vi "Project-SmartHome.vi"() -> ()   [LabVIEW 2013]
uses:
  <vilib>/regexp/Match Regular Expression.xnode
panel:
  in  "Back":bool
  out "Numeric":dbl
  in  "Tab Control 25":enum32{"Page 1", "Page 2"}(tab)
  in  "Back 22":bool
  in  "edit":bool
  out "Table Control":string[][](table)
  in  "String":string
  in  "flag 8":u16(ring) items=["Admin", "User"]
  in  "String":string
  in  "String":string
  in  "delete":bool
  in  "add":bool
  out "channel":dbl
  out "URL":string="C:\\Users\\kiat\\Downloads\\asd.mp4"
  in  "Tab Control 24":enum32{"Page 1", "Page 2"}(tab)
  in  "Back 21":bool
  in  "WindowsMediaPlayer":refnum<k7>(container)
  in  "backward":bool
  in  "foward":bool
  in  "pause":bool
  in  "stop":bool
  in  "flag 7":u16(ring) items=["1", "2", "3"]
  in  "play":bool
  in  "?":dbl(slide) scale=0.0..100.0
  in  "Tab Control 23":enum32{"Page 1", "Page 2"}(tab)
  in  "Back 19":bool
  in  "?":bool
  in  "String":string
  in  "?":bool
  in  "?":dbl(slide) scale=16.0..27.0
  in  "Tab Control 22":enum32{"Page 1", "Page 2"}(tab)
  in  "Back 18":bool
  in  "?":bool
  in  "String":string
  in  "?":bool
  in  "?":dbl(slide) scale=16.0..27.0
  in  "Tab Control 21":enum32{"Page 1", "Page 2"}(tab)
  in  "Back 20":bool
  in  "?":bool
  in  "String":string
  in  "?":bool
  in  "?":dbl(slide) scale=16.0..27.0
  in  "Tab Control 19":enum32{"Page 1", "Page 2"}(tab)
  in  "Back 17":bool
  in  "?":bool
  in  "?":bool
  in  "?":bool
  in  "Tab Control 18":enum32{"Page 1", "Page 2"}(tab)
  in  "Back 12":bool
  in  "?":bool
  in  "start hour 3":u16(ring) items=["1", "2", "3", "4", "5", "6", "7", "8", "9", "10", "11", "12"]
  in  "flag 6":u16(ring) items=["AM", "PM"]
  in  "start min 3":u16(ring) items=["0", "1", "2", "3", "4", "5", "6", "7", "8", "9", "10", "11", "12", "13", "14", "15", "16", "17", "18", "19", "20", "21", "22", "23", "24", "25", "26", "27", "28", "29", "30", "31", "32", "33", "34", "35", "36", "37", "38", "39", "40", "41", "42", "43", "44", "45", "46", "47", "48", "49", "50", "51", "52", "53", "54", "55", "56", "57", "58", "59"]
  in  "end hour 3":u16(ring) items=["1", "2", "3", "4", "5", "6", "7", "8", "9", "10", "11", "12"]
  in  "end min 3":u16(ring) items=["0", "1", "2", "3", "4", "5", "6", "7", "8", "9", "10", "11", "12", "13", "14", "15", "16", "17", "18", "19", "20", "21", "22", "23", "24", "25", "26", "27", "28", "29", "30", "31", "32", "33", "34", "35", "36", "37", "38", "39", "40", "41", "42", "43", "44", "45", "46", "47", "48", "49", "50", "51", "52", "53", "54", "55", "56", "57", "58", "59"]
  in  "flag 5":u16(ring) items=["AM", "PM"]
  in  "String":string
  in  "?":bool
  in  "?":dbl(slide) scale=0.0..4.0
  in  "Tab Control 17":enum32{"Page 1", "Page 2"}(tab)
  in  "Back 11":bool
  in  "flag 3":u16(ring) items=["AM", "PM"]
  in  "end min 2":u16(ring) items=["0", "1", "2", "3", "4", "5", "6", "7", "8", "9", "10", "11", "12", "13", "14", "15", "16", "17", "18", "19", "20", "21", "22", "23", "24", "25", "26", "27", "28", "29", "30", "31", "32", "33", "34", "35", "36", "37", "38", "39", "40", "41", "42", "43", "44", "45", "46", "47", "48", "49", "50", "51", "52", "53", "54", "55", "56", "57", "58", "59"]
  in  "end hour 2":u16(ring) items=["1", "2", "3", "4", "5", "6", "7", "8", "9", "10", "11", "12"]
  in  "start min 2":u16(ring) items=["0", "1", "2", "3", "4", "5", "6", "7", "8", "9", "10", "11", "12", "13", "14", "15", "16", "17", "18", "19", "20", "21", "22", "23", "24", "25", "26", "27", "28", "29", "30", "31", "32", "33", "34", "35", "36", "37", "38", "39", "40", "41", "42", "43", "44", "45", "46", "47", "48", "49", "50", "51", "52", "53", "54", "55", "56", "57", "58", "59"]
  in  "flag 4":u16(ring) items=["AM", "PM"]
  in  "start hour 2":u16(ring) items=["1", "2", "3", "4", "5", "6", "7", "8", "9", "10", "11", "12"]
  in  "?":bool
  in  "String":string
  in  "?":bool
  in  "?":dbl(slide) scale=0.0..4.0
  in  "Tab Control 16":enum32{"Page 1", "Page 2"}(tab)
  in  "Back 9":bool
  in  "?":bool
  in  "?":bool
  in  "?":bool
  in  "Tab Control 15":enum32{"Page 1", "Page 2"}(tab)
  in  "Back 16":bool
  in  "OK Button 32":bool
  in  "OK Button 31":bool
  in  "?":bool
  in  "Tab Control 14":enum32{"Page 1", "Page 2"}(tab)
  in  "Back 15":bool
  in  "OK Button 27":bool
  in  "OK Button 26":bool
  in  "OK Button 25":bool
  in  "?":bool
  in  "Tab Control 13":enum32{"Page 1", "Page 2"}(tab)
  in  "Back 14":bool
  in  "OK Button 24":bool
  in  "OK Button 23":bool
  in  "OK Button 22":bool
  in  "OK Button 21":bool
  in  "OK Button 20":bool
  in  "OK Button 19":bool
  in  "?":bool
  in  "Tab Control 12":enum32{"Page 1", "Page 2"}(tab)
  in  "Back 13":bool
  in  "?":bool
  in  "?":bool
  in  "?":bool
  in  "Tab Control 11":enum32{"Page 1", "Page 2"}(tab)
  in  "Back 10":bool
  in  "flag":u16(ring) items=["AM", "PM"]
  in  "end min 1":u16(ring) items=["0", "1", "2", "3", "4", "5", "6", "7", "8", "9", "10", "11", "12", "13", "14", "15", "16", "17", "18", "19", "20", "21", "22", "23", "24", "25", "26", "27", "28", "29", "30", "31", "32", "33", "34", "35", "36", "37", "38", "39", "40", "41", "42", "43", "44", "45", "46", "47", "48", "49", "50", "51", "52", "53", "54", "55", "56", "57", "58", "59"]
  in  "end hour 1":u16(ring) items=["1", "2", "3", "4", "5", "6", "7", "8", "9", "10", "11", "12"]
  in  "start min 1":u16(ring) items=["0", "1", "2", "3", "4", "5", "6", "7", "8", "9", "10", "11", "12", "13", "14", "15", "16", "17", "18", "19", "20", "21", "22", "23", "24", "25", "26", "27", "28", "29", "30", "31", "32", "33", "34", "35", "36", "37", "38", "39", "40", "41", "42", "43", "44", "45", "46", "47", "48", "49", "50", "51", "52", "53", "54", "55", "56", "57", "58", "59"]
  in  "flag 2":u16(ring) items=["AM", "PM"]
  in  "start hour 1":u16(ring) items=["1", "2", "3", "4", "5", "6", "7", "8", "9", "10", "11", "12"]
  in  "?":bool
  in  "String":string
  in  "?":bool
  in  "?":dbl(slide) scale=0.0..4.0
  in  "Tab Control 10":enum32{"Page 1", "Page 2"}(tab)
  in  "Tab Control 9":enum32{"Page 1", "Page 2"}(tab)
  in  "Back 8":bool
  in  "OK Button 18":bool
  in  "?":bool
  in  "Tab Control 8":enum32{"Page 1", "Page 2"}(tab)
  in  "Back 7":bool
  in  "OK Button 17":bool
  in  "?":bool
  in  "Tab Control 7":enum32{"Page 1", "Page 2"}(tab)
  in  "Back 6":bool
  in  "OK Button 16":bool
  in  "?":bool
  in  "Tab Control 6":enum32{"Page 1", "Page 2"}(tab)
  in  "Back 5":bool
  in  "OK Button 15":bool
  in  "?":bool
  in  "Tab Control 5":enum32{"Page 1", "Page 2"}(tab)
  in  "Back 4":bool
  in  "OK Button 14":bool
  in  "OK Button 13":bool
  in  "OK Button 12":bool
  in  "OK Button 11":bool
  in  "?":bool
  in  "Tab Control 4":enum32{"Page 1", "Page 2"}(tab)
  in  "Back 3":bool
  in  "OK Button 10":bool
  in  "OK Button 9":bool
  in  "OK Button 8":bool
  in  "OK Button 7":bool
  in  "OK Button 6":bool
  in  "OK Button 5":bool
  in  "?":bool
  in  "stop":bool
  in  "Tab Control 3":enum32{"Page 1", "Page 2"}(tab)
  in  "Back 2":bool
  in  "?":bool
  in  "?":bool
  in  "?":bool
  in  "?":bool
  in  "?":bool
  in  "?":bool
  in  "Tab Control 2":enum32{"Page 1"}(tab)
  in  "OK Button 3":bool
  in  "?":bool
  in  "?":bool
  in  "?":bool
  in  "?":bool
  in  "?":bool
  in  "?":bool
  in  "Tab Control":enum32{"Page 1", "Page 2"}(tab)
  in  "String 2":string caption="String"
  in  "OK Button":bool
  in  "String":string
  # "Master room \nlight 1"
  # "Master room \ndoor 1"
  # "Master room \nldoor 1"
  # "Open Area \nlight 1"
  # "Garrden \nlight 1"
  # "Living room \nlight 1"
  # "Living room \nlight 1"
  # "Master bathroom \nlight 1"
  # "Master room \nlight 1"
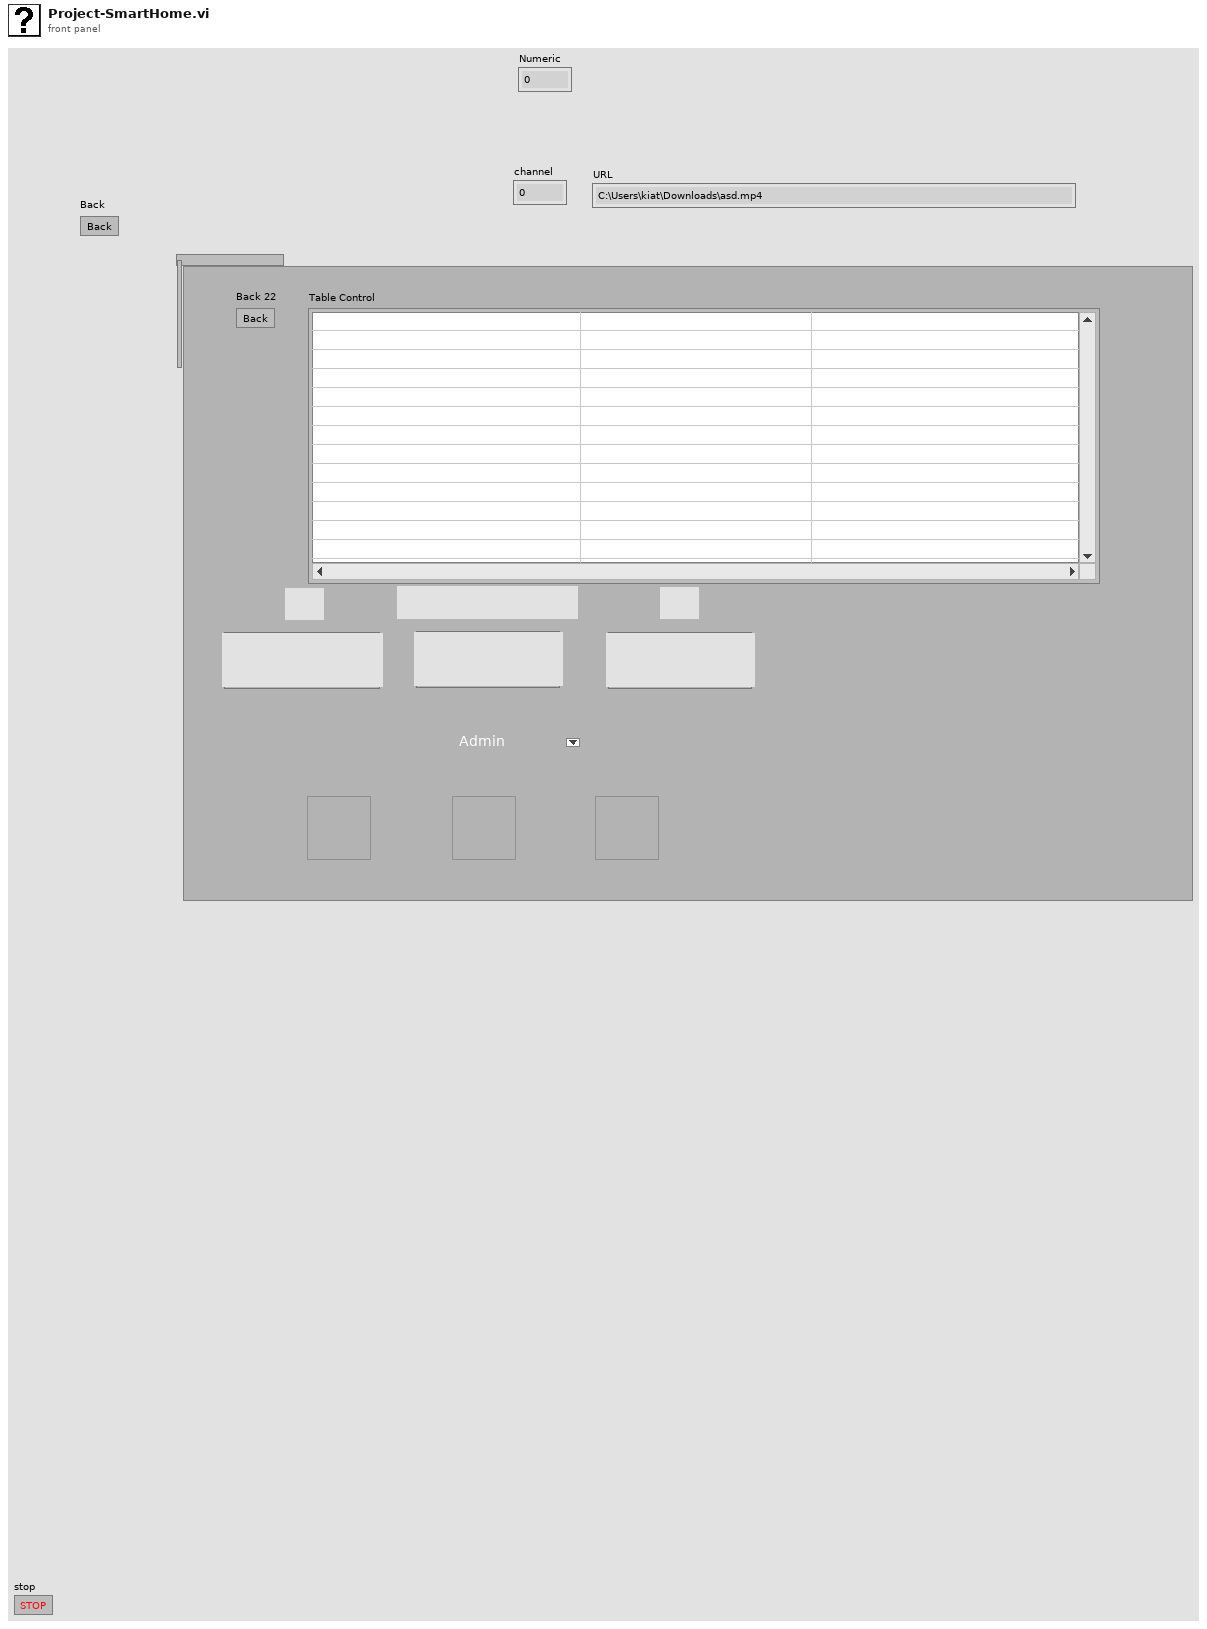
[diagram p1: front panel]
types:
  T1 = enum8{"Enabled", "Disabled", "Disabled and Grayed Out"}
  T2 = enum16{"open", "replace", "create", "open or create", "replace or create", "replace or create with confirmation"}
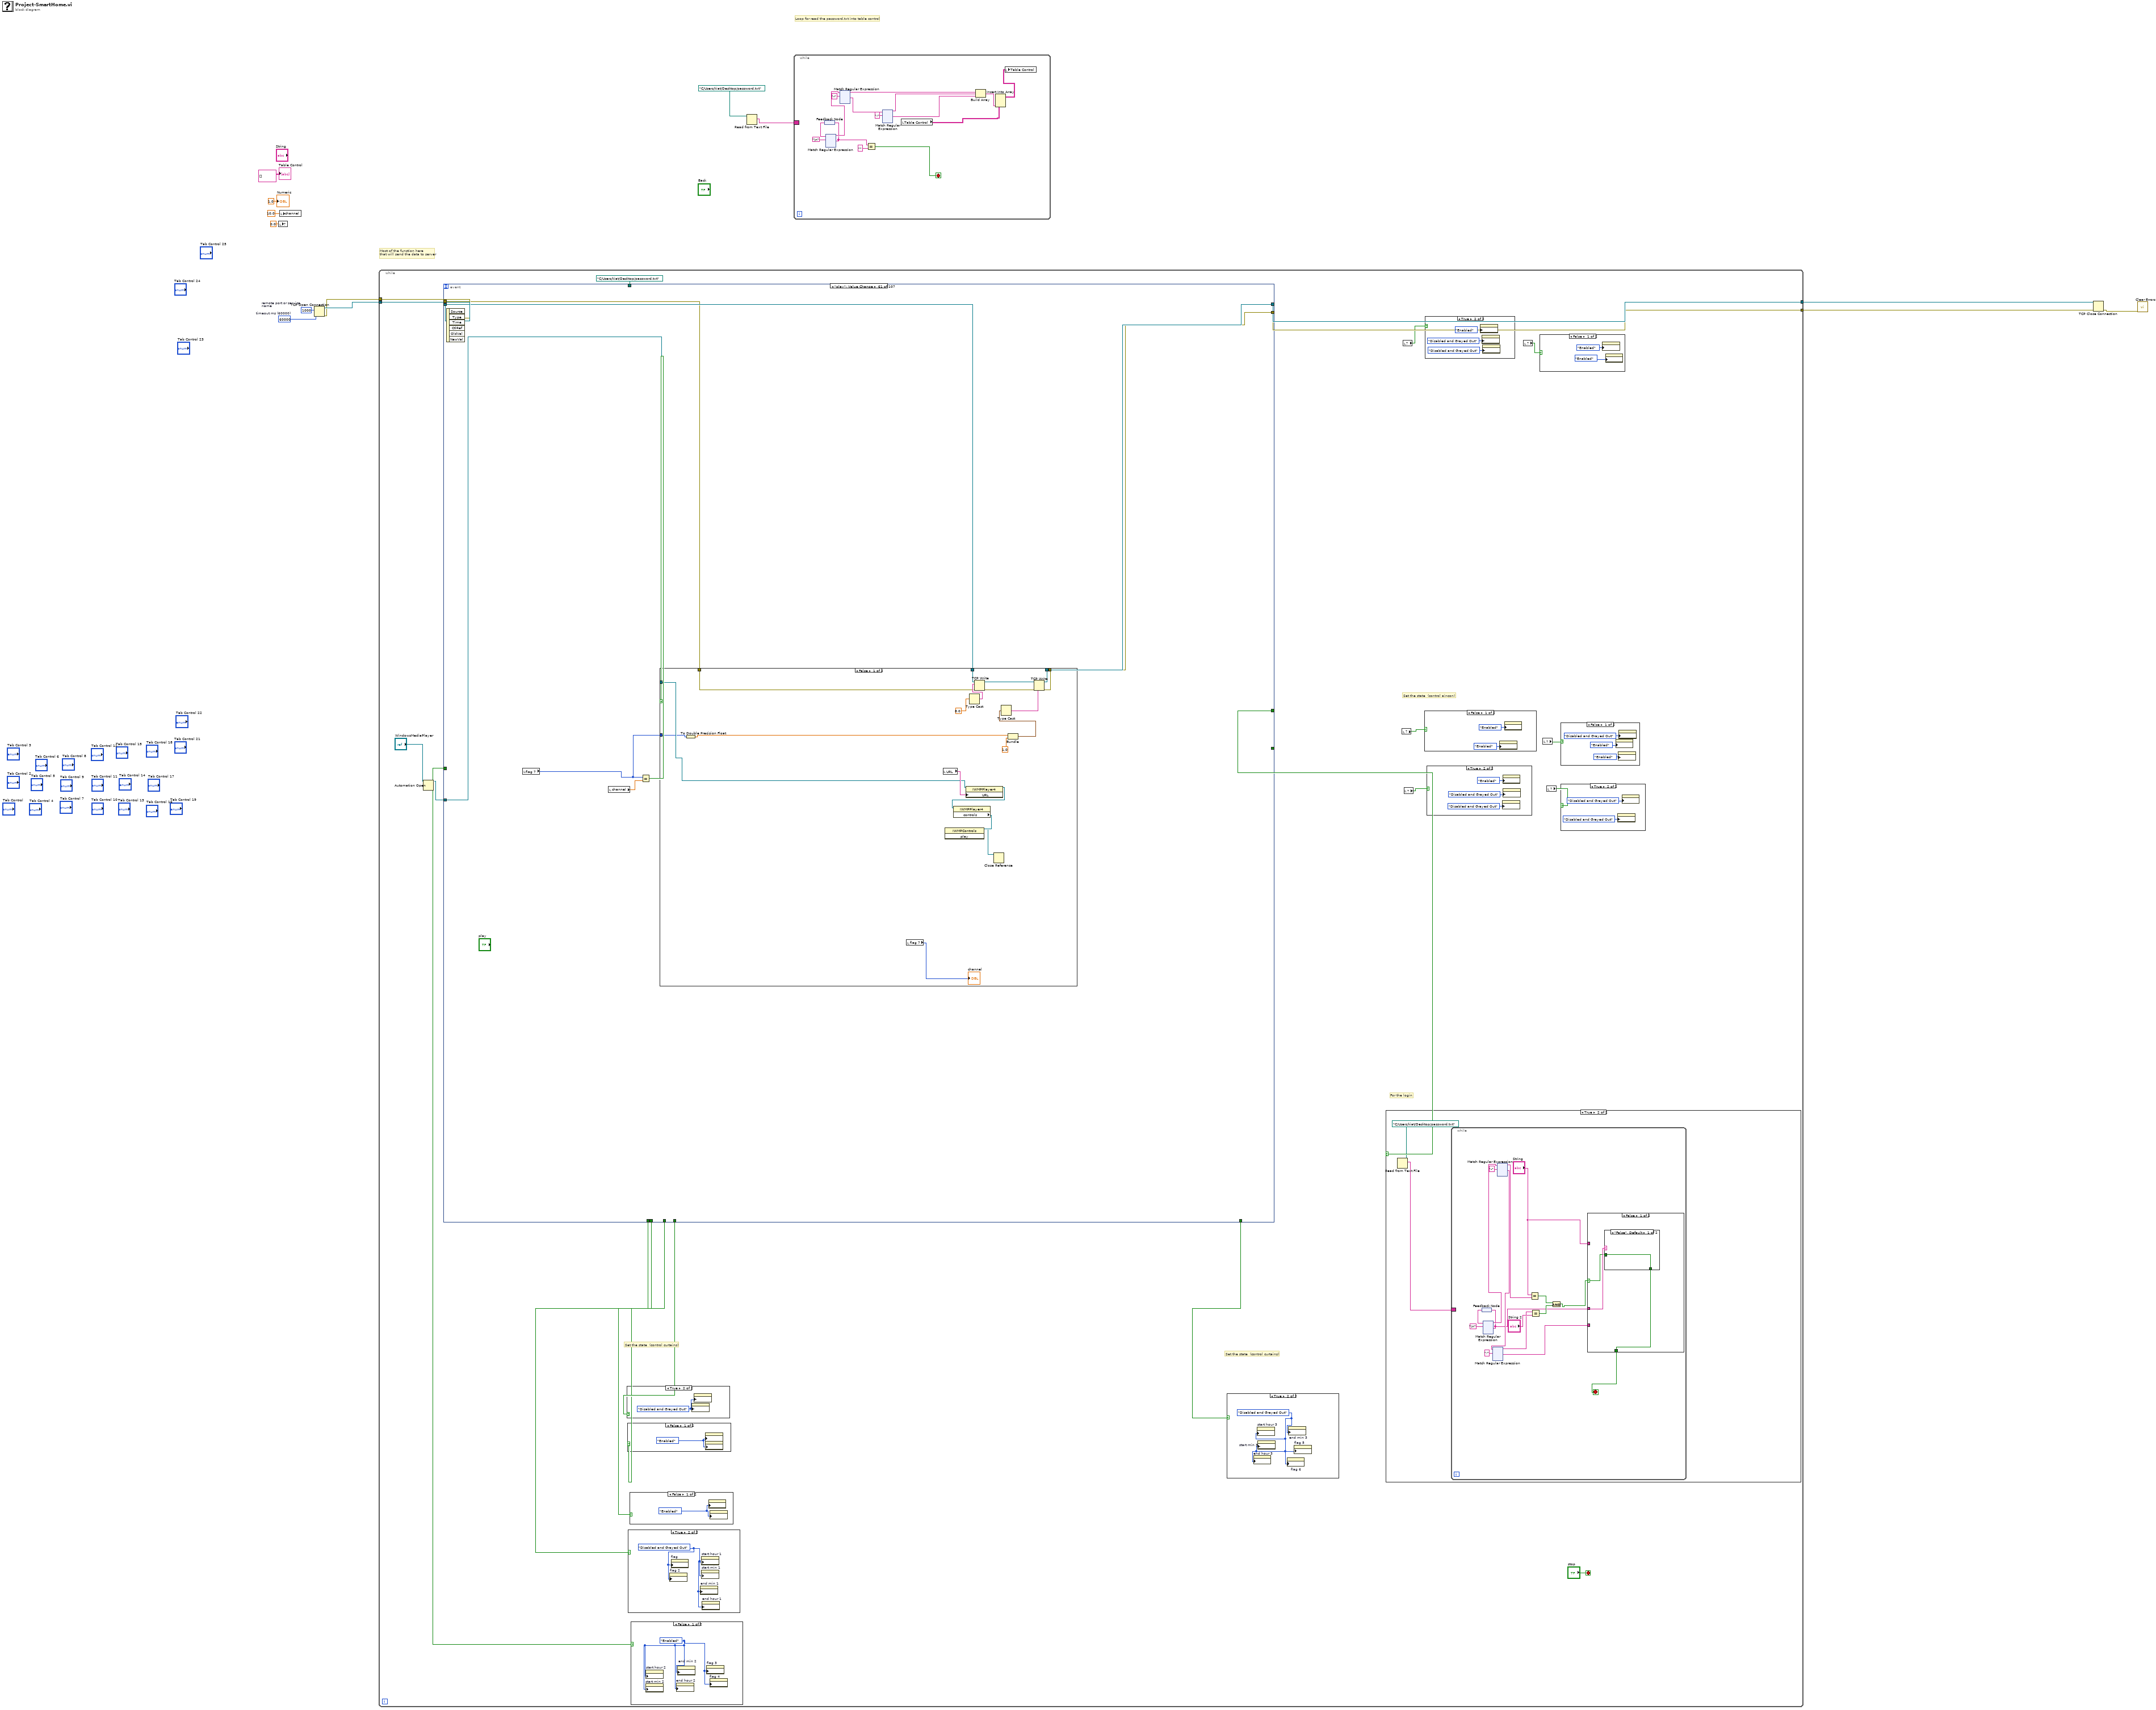
[diagram p0: block diagram]
diagram:
  w12 = 60000  # timeout ms (60000)
  w13 = u16 1000  # remote port or service name
  # "Most of the function here\nthat will send the data to server"
  # "Loop for read the password.txt into table control"
  n1 = local write item#?(0.0) -> ()
  n2 = local write "channel"(10.0 ("Numeric 2")) -> ()
  n3 = TCP Open Connection(remote port or service name=w13, timeout ms (60000)=w12) -> (connection ID=w9:refnum<k5>, error out=w8:errorcluster)  [unwired: 3 in]
  n4 = while {
    tunnel: w9 -> [w33]
    tunnel: w8 -> [w32]
    tunnel: [w30] -> w10
    tunnel: [w29] -> w7
    stop <- "stop" stop-if-true
    # "Set the state  (control air-con)"
    # "Set the state  (control curtains)"
    # "Set the state  (control curtains)"
    # "For the login"
    n5 = Automation Open(Automation Refnum="WindowsMediaPlayer") -> (Automation Refnum=w15:refnum<k7>)  [unwired: 3 in, 1 out]
    n6 = event shown="[60] \"play\": Value Change" {
      selector: _ -> [_ _ _ _ _ _ _ _ _ _ _ _ _ _ _ _ _ _ _ _ _ _ _ _ _ _ _ _ _ _ _ _ _ _ _ _ _ _ _ _ _ _ _ _ _ _ _ _ _ _ _ _ _ _ _ _ _ _ _ _ _ _ _ _ _ _ _ _ _ _ _ _ _ _ _ _ _ _ _ _ _ _ _ _ _ _ _ _ _ _ _ _ _ _ _ _ _ _ _ _ _ _ _ _ _ _ _]
      dyn-events: _ -> [_ _ _ _ _ _ _ _ _ _ _ _ _ _ _ _ _ _ _ _ _ _ _ _ _ _ _ _ _ _ _ _ _ _ _ _ _ _ _ _ _ _ _ _ _ _ _ _ _ _ _ _ _ _ _ _ _ _ _ _ _ _ _ _ _ _ _ _ _ _ _ _ _ _ _ _ _ _ _ _ _ _ _ _ _ _ _ _ _ _ _ _ _ _ _ _ _ _ _ _ _ _ _ _ _ _ _]
      timeout: _ -> [_ _ _ _ _ _ _ _ _ _ _ _ _ _ _ _ _ _ _ _ _ _ _ _ _ _ _ _ _ _ _ _ _ _ _ _ _ _ _ _ _ _ _ _ _ _ _ _ _ _ _ _ _ _ _ _ _ _ _ _ _ _ _ _ _ _ _ _ _ _ _ _ _ _ _ _ _ _ _ _ _ _ _ _ _ _ _ _ _ _ _ _ _ _ _ _ _ _ _ _ _ _ _ _ _ _ _]
      tunnel: [_ "OK Button" _ _ _ _ _ _ _ _ _ _ _ _ _ _ _ _ _ _ _ _ _ _ _ _ _ _ _ _ _ _ _ _ _ _ _ _ _ _ _ _ _ _ _ _ _ _ _ _ _ _ _ _ _ _ _ _ _ _ _ _ _ _ _ _ _ _ _ _ _ _ _ _ _ _ _ _ _ _ _ _ _ _ _ _ _ _ _ _ _ _ _ _ _ _ _ _ _ _ _ _ _ _ _ _ _] -> w34
      tunnel: w33 -> [_ _ _ _ _ w511 w523 _ _ w581 w590 _ w628 w643 w658 w668 w680 _ w713 w728 w741 _ w778 _ _ _ _ _ _ w842 _ _ w900 w911 w923 w937 _ _ _ _ _ _ _ _ _ _ _ _ _ _ _ _ _ _ _ _ w1068 w1079 w1096 _ w1133 _ w1176 w1191 w1203 _ _ _ w2638 _ w2675 w2689 w2703 _ w2740 w2750 w2762 w2774 w2787 w2799 w2812 w2823 w2837 w2850 w2858 w2869 w2884 w2896 _ w2927 w2940 w2953 w2965 w2975 w2986 w3000 w3028 w3058 w3088 _ w3118 _ _ w3177 w3187 w3200 w3214]
      tunnel: [_ _ _ _ _ w517 w529 _ _ w584 w598 _ w630 w642 w656 w674 w686 _ w721 w733 w742 _ w776 _ _ _ _ _ _ w843 _ _ w904 w912 w922 w939 _ _ _ _ _ _ _ _ _ _ _ _ _ _ _ _ _ _ _ _ w1070 w1082 w1093 _ w1131 _ w1174 w1189 w1206 _ _ _ w2636 _ w2673 w2688 w2706 _ w2745 w2758 w2765 w2781 w2792 w2806 w2817 w2829 w2841 w2848 w2864 w2877 w2889 w2901 _ w2933 w2945 w2957 w2969 w2981 w2996 w3004 w3030 w3059 w3089 _ w3122 _ _ w3181 w3193 w3205 w3217] -> w30
      tunnel: w32 -> [_ _ _ _ _ w512 w524 _ _ w582 w593 _ w627 w644 w657 w669 w681 _ w716 w725 w740 _ w777 _ _ _ _ _ _ w841 _ _ w899 w910 w924 w936 _ _ _ _ _ _ _ _ _ _ _ _ _ _ _ _ _ _ _ _ w1067 w1080 w1095 _ w1132 _ w1175 w1190 w1204 _ _ _ w2637 _ w2674 w2690 w2704 _ w2737 w2749 w2763 w2775 w2788 w2800 w2811 w2822 w2836 w2849 w2857 w2872 w2883 w2893 _ w2928 w2941 w2950 w2962 w2974 w2985 w3001 w3027 w3057 w3087 _ w3119 _ _ w3174 w3186 w3199 w3213]
      tunnel: [_ _ _ _ _ w516 w528 _ _ w585 w597 _ w629 w641 w655 w673 w685 _ w720 w732 w743 _ w775 _ _ _ _ _ _ w844 _ _ w903 w913 w921 w938 _ _ _ _ _ _ _ _ _ _ _ _ _ _ _ _ _ _ _ _ w1069 w1081 w1092 _ w1130 _ w1173 w1188 w1205 _ _ _ w2635 _ w2672 w2687 w2705 _ w2744 w2757 w2764 w2782 w2793 w2805 w2816 w2828 w2840 w2847 w2863 w2876 w2888 w2900 _ w2932 w2944 w2958 w2970 w2982 w2995 w3003 w3031 w3060 w3090 _ w3123 _ _ w3182 w3194 w3206 w3218] -> w29
      tunnel: [_ _ _ _ _ _ _ _ _ _ _ _ _ _ _ _ _ _ _ _ _ _ _ _ _ _ _ _ _ _ _ _ _ _ _ "?" _ _ _ _ _ _ _ _ _ _ _ _ _ _ _ _ _ _ _ _ _ _ _ _ _ _ _ _ _ _ _ _ _ _ _ _ _ _ _ _ _ _ _ _ _ _ _ _ _ _ _ _ _ _ _ _ _ _ _ _ _ _ _ _ _ _ _ _ _ _ _] -> w28
      tunnel: [_ _ _ _ _ _ _ _ _ _ _ _ _ _ _ _ _ _ _ _ _ _ _ _ _ _ _ _ _ "?" _ _ _ _ _ _ _ _ _ _ _ _ _ _ _ _ _ _ _ _ _ _ _ _ _ _ _ _ _ _ _ _ _ _ _ _ _ _ _ _ _ _ _ _ _ _ _ _ _ _ _ _ _ _ _ _ _ _ _ _ _ _ _ _ _ _ _ _ _ _ _ _ _ _ _ _ _] -> w27
      tunnel: [_ _ _ _ _ _ _ _ _ _ _ _ _ _ _ _ _ _ _ _ "?" _ _ _ _ _ _ _ _ _ _ _ _ _ _ _ _ _ _ _ _ _ _ _ _ _ _ _ _ _ _ _ _ _ _ _ _ _ _ _ _ _ _ _ _ _ _ _ _ _ _ _ _ _ _ _ _ _ _ _ _ _ _ _ _ _ _ _ _ _ _ _ _ _ _ _ _ _ _ _ _ _ _ _ _ _ _] -> w26
      tunnel: [_ _ _ _ _ _ _ _ _ _ _ _ _ _ _ _ _ _ _ _ _ _ _ _ _ _ _ _ _ _ _ _ _ _ _ _ _ _ _ _ _ _ _ _ _ _ _ _ _ _ _ _ _ _ _ _ _ _ _ _ _ _ _ _ _ _ _ _ _ _ _ _ _ _ _ _ _ _ _ _ _ _ _ _ _ _ _ _ _ _ _ _ _ _ _ _ "?" _ _ _ _ _ _ _ _ _ _] -> w25
      tunnel: [_ _ _ _ _ _ _ _ _ _ _ _ _ _ _ _ _ _ _ _ _ _ _ _ _ _ _ _ _ _ _ _ _ _ _ _ _ _ _ _ _ _ _ _ _ _ _ _ _ _ _ _ _ _ _ _ _ _ _ _ _ _ _ _ _ _ _ _ _ _ _ _ _ _ _ _ _ _ _ _ _ _ _ _ _ _ _ _ _ _ _ _ _ _ _ _ _ "?" _ _ _ _ _ _ _ _ _] -> w24
      tunnel: [_ _ _ _ _ _ _ _ _ _ _ _ _ _ _ _ _ _ _ _ _ _ _ _ _ _ _ _ _ _ _ _ _ _ _ _ _ _ _ _ _ _ _ _ _ _ _ _ _ _ _ _ _ _ _ _ _ _ _ _ _ _ _ _ _ _ _ _ _ _ _ _ _ _ _ _ _ _ _ _ _ _ _ _ _ _ _ _ _ _ _ _ _ _ _ _ _ _ "?" _ _ _ _ _ _ _ _] -> w23
      tunnel: [_ _ _ _ _ _ _ _ _ _ _ _ _ w639 _ _ _ _ _ _ _ _ _ _ _ _ _ _ _ _ _ _ _ _ _ _ _ _ _ _ _ _ _ _ _ _ _ _ _ _ _ _ _ _ _ _ _ _ _ _ _ _ _ _ _ _ _ _ _ _ _ _ _ _ _ _ _ _ _ _ _ _ _ _ _ _ _ _ _ _ _ _ _ _ _ _ _ _ _ _ _ _ _ _ _ _ _] -> _
      tunnel: w15 -> [_ _ _ _ _ _ _ _ _ _ _ _ _ _ _ _ _ _ _ _ _ _ _ _ _ _ _ _ _ _ _ _ _ _ _ _ _ _ _ _ _ _ _ _ _ _ _ _ _ _ _ _ _ _ _ _ _ _ _ _ w1134 _ w1185 w1200 w1215 _ _ _ w2646 _ w2684 _ _ _ _ _ _ _ _ _ _ _ _ _ _ _ _ _ _ _ _ _ _ _ _ _ _ _ _ _ _ _ _ _ _ _ _]
      tunnel: path "C:/Users/kiat/Desktop/password.txt" ("file (use dialog)") -> [_ _ _ _ _ _ _ _ _ _ _ _ _ _ _ _ _ _ _ _ _ _ _ _ _ _ _ _ _ _ _ _ _ _ _ _ _ _ _ _ _ _ _ _ _ _ _ _ _ _ _ _ _ _ _ _ _ _ _ _ _ _ _ _ _ w1219 w1493 w2249 _ _ _ _ _ _ _ _ _ _ _ _ _ _ _ _ _ _ _ _ _ _ _ _ _ _ _ _ _ _ _ _ _ _ _ _ _ _ _]
      event Timeout {
        n7 = event-data() -> ()  [unwired: 1 in, 3 out]
      }
      event "OK Button": Value Change {
        n8 = event-data() -> ()  [unwired: 1 in, 6 out]
      }
      event "Back 2": Value Change {
        n9 = event-data() -> ()  [unwired: 1 in, 6 out]
        n10 = property on="Tab Control 3" class="TabCtl (strict)"("Visible"=FALSE) -> ()  [unwired: 2 in, 2 out]
        n11 = property on="Tab Control 2" class="TabCtl (strict)"("Visible"=TRUE) -> ()  [unwired: 2 in, 2 out]
        n12 = property on="Tab Control" class="TabCtl (strict)"("Visible"=FALSE) -> ()  [unwired: 2 in, 2 out]
      }
      event "OK Button 3": Value Change {
        w461 = TRUE
        n13 = event-data() -> ()  [unwired: 1 in, 6 out]
        n14 = property on="Tab Control 5" class="TabCtl (strict)"("Visible"=FALSE) -> ()  [unwired: 2 in, 2 out]
        n15 = property on="Tab Control 3" class="TabCtl (strict)"("Visible"=FALSE) -> ()  [unwired: 2 in, 2 out]
        n16 = property on="Tab Control 21" class="TabCtl (strict)"("Visible"=FALSE) -> ()  [unwired: 2 in, 2 out]
        n17 = property on="Tab Control 9" class="TabCtl (strict)"("Visible"=FALSE) -> ()  [unwired: 2 in, 2 out]
        n18 = property on="Tab Control 22" class="TabCtl (strict)"("Visible"=FALSE) -> ()  [unwired: 2 in, 2 out]
        n19 = property on="Tab Control 23" class="TabCtl (strict)"("Visible"=FALSE) -> ()  [unwired: 2 in, 2 out]
        n20 = property on="Tab Control 4" class="TabCtl (strict)"("Visible"=FALSE) -> ()  [unwired: 2 in, 2 out]
        n21 = property on="Tab Control 12" class="TabCtl (strict)"("Visible"=FALSE) -> ()  [unwired: 2 in, 2 out]
        n22 = property on="Tab Control 19" class="TabCtl (strict)"("Visible"=FALSE) -> ()  [unwired: 2 in, 2 out]
        n23 = property on="Tab Control 24" class="TabCtl (strict)"("Visible"=FALSE) -> ()  [unwired: 2 in, 2 out]
        n24 = property on="Tab Control 7" class="TabCtl (strict)"("Visible"=FALSE) -> ()  [unwired: 2 in, 2 out]
        n25 = property on="Tab Control 14" class="TabCtl (strict)"("Visible"=FALSE) -> ()  [unwired: 2 in, 2 out]
        n26 = property on="Tab Control 16" class="TabCtl (strict)"("Visible"=FALSE) -> ()  [unwired: 2 in, 2 out]
        n27 = property on="Tab Control 13" class="TabCtl (strict)"("Visible"=FALSE) -> ()  [unwired: 2 in, 2 out]
        n28 = property on="Tab Control 25" class="TabCtl (strict)"("Visible"=FALSE) -> ()  [unwired: 2 in, 2 out]
        n29 = property on="Tab Control 15" class="TabCtl (strict)"("Visible"=FALSE) -> ()  [unwired: 2 in, 2 out]
        n30 = property on="Tab Control 8" class="TabCtl (strict)"("Visible"=FALSE) -> ()  [unwired: 2 in, 2 out]
        n31 = property on="Tab Control 10" class="TabCtl (strict)"("Visible"=FALSE) -> ()  [unwired: 2 in, 2 out]
        n32 = property on="Tab Control 6" class="TabCtl (strict)"("Visible"=FALSE) -> ()  [unwired: 2 in, 2 out]
        n33 = property on="Tab Control 11" class="TabCtl (strict)"("Visible"=FALSE) -> ()  [unwired: 2 in, 2 out]
        n34 = property on="Tab Control 2" class="TabCtl (strict)"("Visible"=FALSE) -> ()  [unwired: 2 in, 2 out]
        n35 = property on="Tab Control 18" class="TabCtl (strict)"("Visible"=FALSE) -> ()  [unwired: 2 in, 2 out]
        n36 = property on="Tab Control 17" class="TabCtl (strict)"("Visible"=FALSE) -> ()  [unwired: 2 in, 2 out]
        n37 = property on="Tab Control" class="TabCtl (strict)"("Visible"=TRUE) -> ()  [unwired: 2 in, 2 out]
        n38 = property class="Bool"("Visible"=w461) -> ()  [unwired: 2 in, 2 out]
        n39 = property on="OK Button 5" class="Bool (strict)"("Visible"=w461) -> ()  [unwired: 2 in, 2 out]
        n40 = property class="Bool (strict)"("Visible"=w461) -> ()  [unwired: 2 in, 2 out]
        n41 = property class="Bool"("Visible"=w461) -> ()  [unwired: 2 in, 2 out]
        n42 = property class="Bool"("Visible"=w461) -> ()  [unwired: 2 in, 2 out]
      }
      event Value Change {
        n43 = event-data() -> ()  [unwired: 1 in, 6 out]
        n44 = property on="Tab Control 17" class="TabCtl (strict)"("Visible"=FALSE) -> ()  [unwired: 2 in, 2 out]
        n45 = property on="Tab Control 3" class="TabCtl (strict)"("Visible"=FALSE) -> ()  [unwired: 2 in, 2 out]
        n46 = property on="Tab Control 11" class="TabCtl (strict)"("Visible"=FALSE) -> ()  [unwired: 2 in, 2 out]
        n47 = property on="Tab Control 6" class="TabCtl (strict)"("Visible"=TRUE) -> ()  [unwired: 2 in, 2 out]
        n48 = property on="Tab Control 10" class="TabCtl (strict)"("Visible"=FALSE) -> ()  [unwired: 2 in, 2 out]
        n49 = property on="Tab Control 18" class="TabCtl (strict)"("Visible"=FALSE) -> ()  [unwired: 2 in, 2 out]
        n50 = property on="Tab Control 2" class="TabCtl (strict)"("Visible"=FALSE) -> ()  [unwired: 2 in, 2 out]
        n51 = property on="Tab Control 5" class="TabCtl (strict)"("Visible"=FALSE) -> ()  [unwired: 2 in, 2 out]
        n52 = property on="Tab Control 9" class="TabCtl (strict)"("Visible"=FALSE) -> ()  [unwired: 2 in, 2 out]
        n53 = property on="Tab Control" class="TabCtl (strict)"("Visible"=FALSE) -> ()  [unwired: 2 in, 2 out]
        n54 = property on="Tab Control 8" class="TabCtl (strict)"("Visible"=FALSE) -> ()  [unwired: 2 in, 2 out]
        n55 = property on="Tab Control 22" class="TabCtl (strict)"("Visible"=FALSE) -> ()  [unwired: 2 in, 2 out]
        n56 = property on="Tab Control 12" class="TabCtl (strict)"("Visible"=FALSE) -> ()  [unwired: 2 in, 2 out]
        n57 = property on="Tab Control 4" class="TabCtl (strict)"("Visible"=FALSE) -> ()  [unwired: 2 in, 2 out]
        n58 = property on="Tab Control 23" class="TabCtl (strict)"("Visible"=FALSE) -> ()  [unwired: 2 in, 2 out]
        n59 = property on="Tab Control 19" class="TabCtl (strict)"("Visible"=FALSE) -> ()  [unwired: 2 in, 2 out]
        n60 = property on="Tab Control 7" class="TabCtl (strict)"("Visible"=FALSE) -> ()  [unwired: 2 in, 2 out]
        n61 = property on="Tab Control 14" class="TabCtl (strict)"("Visible"=FALSE) -> ()  [unwired: 2 in, 2 out]
        n62 = property on="Tab Control 13" class="TabCtl (strict)"("Visible"=FALSE) -> ()  [unwired: 2 in, 2 out]
        n63 = property on="Tab Control 15" class="TabCtl (strict)"("Visible"=FALSE) -> ()  [unwired: 2 in, 2 out]
        n64 = property on="Tab Control 24" class="TabCtl (strict)"("Visible"=FALSE) -> ()  [unwired: 2 in, 2 out]
        n65 = property on="Tab Control 21" class="TabCtl (strict)"("Visible"=FALSE) -> ()  [unwired: 2 in, 2 out]
        n66 = property on="Tab Control 16" class="TabCtl (strict)"("Visible"=FALSE) -> ()  [unwired: 2 in, 2 out]
      }
      event Value Change {
        n67 = event-data() -> ()  [unwired: 1 in, 6 out]
        n68 = Type Cast(x=0.0) -> (*(type *) &x=w514:string)  [unwired: 1 in]
        n69 = TCP Write(connection ID=w511, data in=w514, error in (no error)=w512) -> (connection ID out=w510:refnum<k5>, error out=w509:errorcluster)  [unwired: 1 in, 1 out]
        n70 = Bundle("?", 13.0) -> (w515:cluster{bool, dbl})  [unwired: 1 in]
        n71 = Type Cast(x=w515) -> (*(type *) &x=w520:string)  [unwired: 1 in]
        n72 = TCP Write(connection ID=w510, data in=w520, error in (no error)=w509) -> (connection ID out=w517:refnum<k5>, error out=w516:errorcluster)  [unwired: 1 in, 1 out]
      }
      event "OK Button 15": Value Change {
        n73 = event-data() -> ()  [unwired: 1 in, 6 out]
        n74 = Type Cast(x=0.0) -> (*(type *) &x=w526:string)  [unwired: 1 in]
        n75 = TCP Write(connection ID=w523, data in=w526, error in (no error)=w524) -> (connection ID out=w522:refnum<k5>, error out=w521:errorcluster)  [unwired: 1 in, 1 out]
        n76 = Bundle("OK Button 15"="OK Button 15", 12.0) -> (w530:cluster{"OK Button 15":bool, dbl})  [unwired: 1 in]
        n77 = Type Cast(x=w530) -> (*(type *) &x=w532:string)  [unwired: 1 in]
        n78 = TCP Write(connection ID=w522, data in=w532, error in (no error)=w521) -> (connection ID out=w529:refnum<k5>, error out=w528:errorcluster)  [unwired: 1 in, 1 out]
      }
      event Value Change {
        n79 = event-data() -> ()  [unwired: 1 in, 6 out]
        n80 = property on="Tab Control 18" class="TabCtl (strict)"("Visible"=FALSE) -> ()  [unwired: 2 in, 2 out]
        n81 = property on="Tab Control 17" class="TabCtl (strict)"("Visible"=FALSE) -> ()  [unwired: 2 in, 2 out]
        n82 = property on="Tab Control 21" class="TabCtl (strict)"("Visible"=FALSE) -> ()  [unwired: 2 in, 2 out]
        n83 = property on="Tab Control 16" class="TabCtl (strict)"("Visible"=FALSE) -> ()  [unwired: 2 in, 2 out]
        n84 = property on="Tab Control 10" class="TabCtl (strict)"("Visible"=FALSE) -> ()  [unwired: 2 in, 2 out]
        n85 = property on="Tab Control 5" class="TabCtl (strict)"("Visible"=FALSE) -> ()  [unwired: 2 in, 2 out]
        n86 = property on="Tab Control 3" class="TabCtl (strict)"("Visible"=FALSE) -> ()  [unwired: 2 in, 2 out]
        n87 = property on="Tab Control 6" class="TabCtl (strict)"("Visible"=FALSE) -> ()  [unwired: 2 in, 2 out]
        n88 = property on="Tab Control 23" class="TabCtl (strict)"("Visible"=FALSE) -> ()  [unwired: 2 in, 2 out]
        n89 = property on="Tab Control 12" class="TabCtl (strict)"("Visible"=FALSE) -> ()  [unwired: 2 in, 2 out]
        n90 = property on="Tab Control 2" class="TabCtl (strict)"("Visible"=FALSE) -> ()  [unwired: 2 in, 2 out]
        n91 = property on="Tab Control 7" class="TabCtl (strict)"("Visible"=TRUE) -> ()  [unwired: 2 in, 2 out]
        n92 = property on="Tab Control 4" class="TabCtl (strict)"("Visible"=FALSE) -> ()  [unwired: 2 in, 2 out]
        n93 = property on="Tab Control 24" class="TabCtl (strict)"("Visible"=FALSE) -> ()  [unwired: 2 in, 2 out]
        n94 = property on="Tab Control 11" class="TabCtl (strict)"("Visible"=FALSE) -> ()  [unwired: 2 in, 2 out]
        n95 = property on="Tab Control" class="TabCtl (strict)"("Visible"=FALSE) -> ()  [unwired: 2 in, 2 out]
        n96 = property on="Tab Control 8" class="TabCtl (strict)"("Visible"=FALSE) -> ()  [unwired: 2 in, 2 out]
        n97 = property on="Tab Control 9" class="TabCtl (strict)"("Visible"=FALSE) -> ()  [unwired: 2 in, 2 out]
        n98 = property on="Tab Control 22" class="TabCtl (strict)"("Visible"=FALSE) -> ()  [unwired: 2 in, 2 out]
        n99 = property on="Tab Control 14" class="TabCtl (strict)"("Visible"=FALSE) -> ()  [unwired: 2 in, 2 out]
        n100 = property on="Tab Control 13" class="TabCtl (strict)"("Visible"=FALSE) -> ()  [unwired: 2 in, 2 out]
        n101 = property on="Tab Control 15" class="TabCtl (strict)"("Visible"=FALSE) -> ()  [unwired: 2 in, 2 out]
        n102 = property on="Tab Control 19" class="TabCtl (strict)"("Visible"=FALSE) -> ()  [unwired: 2 in, 2 out]
      }
      event Value Change {
        n103 = event-data() -> ()  [unwired: 1 in, 6 out]
        n104 = property on="Tab Control 16" class="TabCtl (strict)"("Visible"=FALSE) -> ()  [unwired: 2 in, 2 out]
        n105 = property on="Tab Control 6" class="TabCtl (strict)"("Visible"=FALSE) -> ()  [unwired: 2 in, 2 out]
        n106 = property on="Tab Control 10" class="TabCtl (strict)"("Visible"=FALSE) -> ()  [unwired: 2 in, 2 out]
        n107 = property on="Tab Control 18" class="TabCtl (strict)"("Visible"=FALSE) -> ()  [unwired: 2 in, 2 out]
        n108 = property on="Tab Control 17" class="TabCtl (strict)"("Visible"=FALSE) -> ()  [unwired: 2 in, 2 out]
        n109 = property on="Tab Control 21" class="TabCtl (strict)"("Visible"=FALSE) -> ()  [unwired: 2 in, 2 out]
        n110 = property on="Tab Control 5" class="TabCtl (strict)"("Visible"=FALSE) -> ()  [unwired: 2 in, 2 out]
        n111 = property on="Tab Control 4" class="TabCtl (strict)"("Visible"=FALSE) -> ()  [unwired: 2 in, 2 out]
        n112 = property on="Tab Control 3" class="TabCtl (strict)"("Visible"=FALSE) -> ()  [unwired: 2 in, 2 out]
        n113 = property on="Tab Control" class="TabCtl (strict)"("Visible"=FALSE) -> ()  [unwired: 2 in, 2 out]
        n114 = property on="Tab Control 2" class="TabCtl (strict)"("Visible"=FALSE) -> ()  [unwired: 2 in, 2 out]
        n115 = property on="Tab Control 12" class="TabCtl (strict)"("Visible"=FALSE) -> ()  [unwired: 2 in, 2 out]
        n116 = property on="Tab Control 22" class="TabCtl (strict)"("Visible"=FALSE) -> ()  [unwired: 2 in, 2 out]
        n117 = property on="Tab Control 7" class="TabCtl (strict)"("Visible"=FALSE) -> ()  [unwired: 2 in, 2 out]
        n118 = property on="Tab Control 11" class="TabCtl (strict)"("Visible"=FALSE) -> ()  [unwired: 2 in, 2 out]
        n119 = property on="Tab Control 8" class="TabCtl (strict)"("Visible"=TRUE) -> ()  [unwired: 2 in, 2 out]
        n120 = property on="Tab Control 9" class="TabCtl (strict)"("Visible"=FALSE) -> ()  [unwired: 2 in, 2 out]
        n121 = property on="Tab Control 14" class="TabCtl (strict)"("Visible"=FALSE) -> ()  [unwired: 2 in, 2 out]
        n122 = property on="Tab Control 13" class="TabCtl (strict)"("Visible"=FALSE) -> ()  [unwired: 2 in, 2 out]
        n123 = property on="Tab Control 15" class="TabCtl (strict)"("Visible"=FALSE) -> ()  [unwired: 2 in, 2 out]
        n124 = property on="Tab Control 24" class="TabCtl (strict)"("Visible"=FALSE) -> ()  [unwired: 2 in, 2 out]
        n125 = property on="Tab Control 23" class="TabCtl (strict)"("Visible"=FALSE) -> ()  [unwired: 2 in, 2 out]
        n126 = property on="Tab Control 19" class="TabCtl (strict)"("Visible"=FALSE) -> ()  [unwired: 2 in, 2 out]
      }
      event Value Change {
        n127 = event-data() -> ()  [unwired: 1 in, 6 out]
        n128 = Type Cast(x=0.0) -> ()  [unwired: 1 in, 1 out]
        n129 = TCP Write(connection ID=w581, error in (no error)=w582) -> (connection ID out=w580:refnum<k5>, error out=w579:errorcluster)  [unwired: 2 in, 1 out]
        n130 = Bundle("?", 17.0) -> (w587:cluster{bool, dbl})  [unwired: 1 in]
        n131 = Type Cast(x=w587) -> (*(type *) &x=w589:string)  [unwired: 1 in]
        n132 = TCP Write(connection ID=w580, data in=w589, error in (no error)=w579) -> (connection ID out=w584:refnum<k5>, error out=w585:errorcluster)  [unwired: 1 in, 1 out]
      }
      event "OK Button 17": Value Change {
        n133 = event-data() -> ()  [unwired: 1 in, 6 out]
        n134 = Type Cast(x=0.0) -> (*(type *) &x=w595:string)  [unwired: 1 in]
        n135 = TCP Write(connection ID=w590, data in=w595, error in (no error)=w593) -> (connection ID out=w591:refnum<k5>, error out=w592:errorcluster)  [unwired: 1 in, 1 out]
        n136 = Bundle("OK Button 17"="OK Button 17", 18.0) -> (w599:cluster{"OK Button 17":bool, dbl})  [unwired: 1 in]
        n137 = Type Cast(x=w599) -> (*(type *) &x=w601:string)  [unwired: 1 in]
        n138 = TCP Write(connection ID=w591, data in=w601, error in (no error)=w592) -> (connection ID out=w598:refnum<k5>, error out=w597:errorcluster)  [unwired: 1 in, 1 out]
      }
      event Value Change {
        n139 = event-data() -> ()  [unwired: 1 in, 6 out]
        n140 = property on="Tab Control 6" class="TabCtl (strict)"("Visible"=FALSE) -> ()  [unwired: 2 in, 2 out]
        n141 = property on="Tab Control 18" class="TabCtl (strict)"("Visible"=FALSE) -> (error out=w607:errorcluster)  [unwired: 2 in, 1 out]
        n142 = property on="Tab Control 17" class="TabCtl (strict)"("Visible"=FALSE) -> ()  [unwired: 2 in, 2 out]
        n143 = property on="Tab Control 21" class="TabCtl (strict)"("Visible"=FALSE) -> ()  [unwired: 2 in, 2 out]
        n144 = property on="Tab Control 10" class="TabCtl (strict)"("Visible"=FALSE) -> ()  [unwired: 2 in, 2 out]
        n145 = property on="Tab Control 12" class="TabCtl (strict)"(error in=w607, "Visible"=FALSE) -> ()  [unwired: 1 in, 2 out]
        n146 = property on="Tab Control 24" class="TabCtl (strict)"("Visible"=FALSE) -> ()  [unwired: 2 in, 2 out]
        n147 = property on="Tab Control 5" class="TabCtl (strict)"("Visible"=FALSE) -> ()  [unwired: 2 in, 2 out]
        n148 = property on="Tab Control 4" class="TabCtl (strict)"("Visible"=FALSE) -> ()  [unwired: 2 in, 2 out]
        n149 = property on="Tab Control 3" class="TabCtl (strict)"("Visible"=FALSE) -> ()  [unwired: 2 in, 2 out]
        n150 = property on="Tab Control" class="TabCtl (strict)"("Visible"=FALSE) -> ()  [unwired: 2 in, 2 out]
        n151 = property on="Tab Control 2" class="TabCtl (strict)"("Visible"=FALSE) -> ()  [unwired: 2 in, 2 out]
        n152 = property on="Tab Control 22" class="TabCtl (strict)"("Visible"=FALSE) -> ()  [unwired: 2 in, 2 out]
        n153 = property on="Tab Control 7" class="TabCtl (strict)"("Visible"=FALSE) -> ()  [unwired: 2 in, 2 out]
        n154 = property on="Tab Control 9" class="TabCtl (strict)"("Visible"=TRUE) -> ()  [unwired: 2 in, 2 out]
        n155 = property on="Tab Control 11" class="TabCtl (strict)"("Visible"=FALSE) -> ()  [unwired: 2 in, 2 out]
        n156 = property on="Tab Control 8" class="TabCtl (strict)"("Visible"=FALSE) -> ()  [unwired: 2 in, 2 out]
        n157 = property on="Tab Control 16" class="TabCtl (strict)"("Visible"=FALSE) -> ()  [unwired: 2 in, 2 out]
        n158 = property on="Tab Control 23" class="TabCtl (strict)"("Visible"=FALSE) -> ()  [unwired: 2 in, 2 out]
        n159 = property on="Tab Control 14" class="TabCtl (strict)"("Visible"=FALSE) -> ()  [unwired: 2 in, 2 out]
        n160 = property on="Tab Control 13" class="TabCtl (strict)"("Visible"=FALSE) -> ()  [unwired: 2 in, 2 out]
        n161 = property on="Tab Control 15" class="TabCtl (strict)"("Visible"=FALSE) -> ()  [unwired: 2 in, 2 out]
        n162 = property on="Tab Control 19" class="TabCtl (strict)"("Visible"=FALSE) -> ()  [unwired: 2 in, 2 out]
      }
      event Value Change {
        # "Air conditional - Bed room (slider)"
        n163 = event-data() -> ()  [unwired: 1 in, 6 out]
        n164 = Type Cast(x=5.0) -> (*(type *) &x=w632:string)  [unwired: 1 in]
        n165 = TCP Write(connection ID=w628, data in=w632, error in (no error)=w627) -> (connection ID out=w634:refnum<k5>, error out=w635:errorcluster)  [unwired: 1 in, 1 out]
        n166 = Bundle("?", "?", 1.0) -> (w636:cluster{bool, dbl, dbl})  [unwired: 1 in]
        n167 = Type Cast(x=w636) -> (*(type *) &x=w638:string)  [unwired: 1 in]
        n168 = TCP Write(connection ID=w634, data in=w638, error in (no error)=w635) -> (connection ID out=w630:refnum<k5>, error out=w629:errorcluster)  [unwired: 1 in, 1 out]
      }
      event Value Change {
        # "Air conditional - Bed room"
        n169 = event-data() -> ()  [unwired: 1 in, 6 out]
        n170 = local read item#9() -> (w639:bool)
        n171 = local read item#12() -> (w640:dbl)
        n172 = Type Cast(x=5.0) -> (*(type *) &x=w645:string)  [unwired: 1 in]
        n173 = TCP Write(connection ID=w643, data in=w645, error in (no error)=w644) -> (connection ID out=w647:refnum<k5>, error out=w648:errorcluster)  [unwired: 1 in, 1 out]
        n174 = Bundle(w639, w640, 1.0) -> (w649:cluster{bool, dbl, dbl})  [unwired: 1 in]
        n175 = Type Cast(x=w649) -> (*(type *) &x=w651:string)  [unwired: 1 in]
        n176 = TCP Write(connection ID=w647, data in=w651, error in (no error)=w648) -> (connection ID out=w642:refnum<k5>, error out=w641:errorcluster)  [unwired: 1 in, 1 out]